vi "45-1523-1 Functional Test.vi"() -> ()   [LabVIEW 2015]
uses:
  <vilib>/DAQmx/write.llb/DAQmx Write (Digital Bool 1Line 1Point).vi
  <vilib>/DAQmx/read.llb/DAQmx Read (Analog DBL 1Chan 1Samp).vi
  Cases.ctl
  <vilib>/ErrorRing/Error Ring.xnode
  <vilib>/LabVIEW Interface for Arduino/LabVIEW Interface for Arduino.lvlib
panel:
  in  "EXIT Button":bool
  in  "Tab Control":T1(tab)
  in  "START Button":bool
  in  "Restart Button":bool
  in  "OK Button":bool
  in  "OK Button 10":bool
  in  "OK Button 3":bool
  in  "OK Button 4":bool
  in  "Restart Button 2":bool
  in  "START Button 2":bool caption="START Button"
  in  "OK Button 5":bool
  in  "OK Button 6":bool
  in  "OK Button 7":bool
  in  "OK Button 8":bool
  in  "OK Button 9":bool
  in  "OK Button 11":bool
  in  "OK Button 12":bool
  # "45-1523-1 Functional Tester"
  # "Click \"START TEST\" To Begin Test"
  # "TESTING J15..."
  # "TESTING K2..."
  # "TESTING K3..."
  # "TESTING K4..."
  # "ALL TESTS PASSED!"
  # "CHECK HIGHLIGHTED CONNECTIONS"
  # "SWITCH K2 FAILED!"
  # "SWITCH K3 FAILED!"
  # "SWITCH K4 FAILED!"
  # "Test Failed"
  # "Verify Connections, then Click \"START\""
  # "Possible Locations of Failure:\n   - Switch K1\n   - S1 Jumper\n   - Q4\n   - U1\n   - Q5"
  # "CHECK HIGHLIGHTED CONNECTIONS"
  # "Power Fault to Board"
  # "CHECK HIGHLIGHTED CONNECTION"
  # "Are All Three LEDs Lit?"
  # "Possible Causes of Failure:\n   - LEDs (Reversed or Faulty)\n   - U1\n   - Q2"
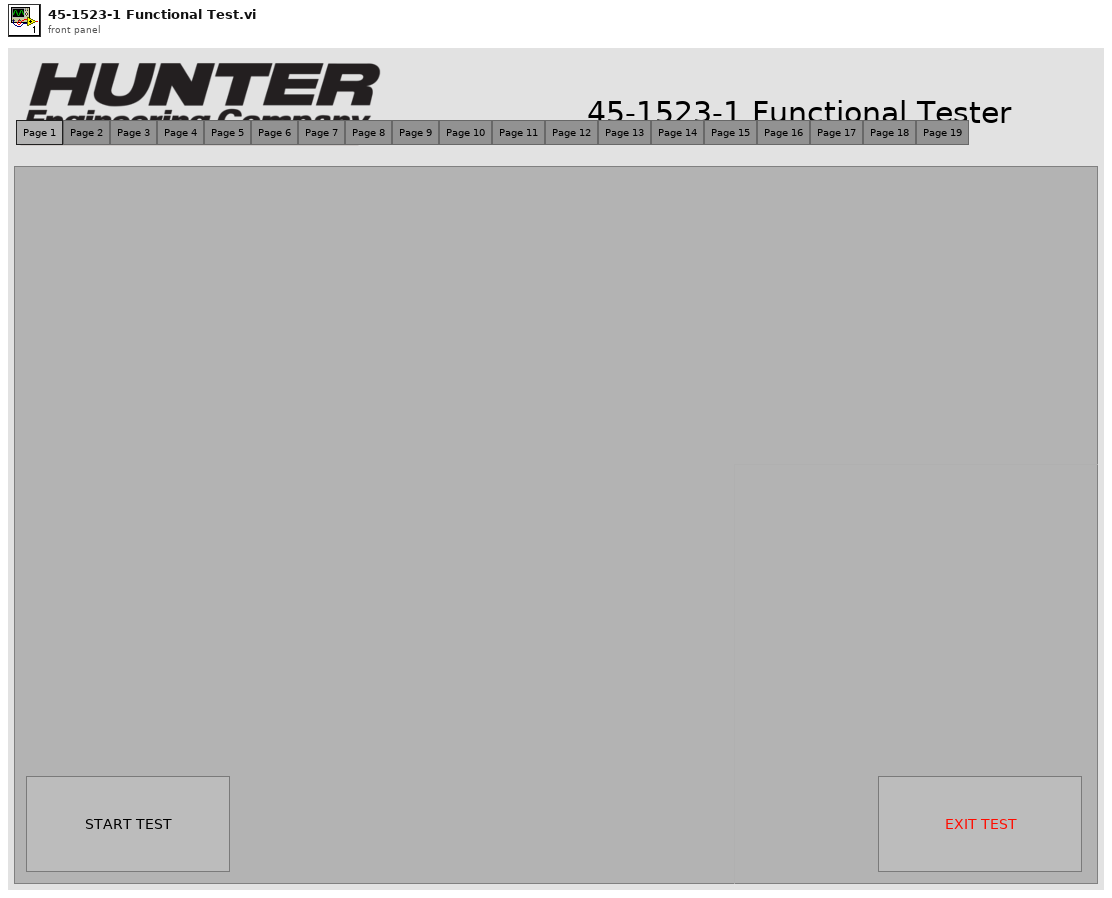
[diagram p1: front panel]
types:
  T1 = enum32{"Page 1", "Page 2", "Page 3", "Page 4", "Page 5", "Page 6", "Page 7", "Page 8", "Page 9", "Page 10", "Page 11", "Page 12", "Page 13", "Page 14", "Page 15", "Page 16", "Page 17", "Page 18", "Page 19"}
  T2 = typedef "Cases.ctl" = enum16{"Start", "Initalization", "J16 Test", "J15 Test", "J15 Error Page", "K2 Test", "K2 Error Page", "K3 Test", "K3 Error Page", "K4 Test", "K4 Error Page", "Test Complete", "Test Failed", "Error", "J15 Failed", "J16 Error", "J16 Failed", "K2 Failed", "LEDs Failed"}
  T3 = typedef "LabVIEW Interface for Arduino.lvlib/Arduino Resource.ctl" = cluster{"VISA resource":refnum<visa-resource-name>, "Board Type":T4, "Connection Type":enum8{"USB / Serial"}, "Bytes Per Packet (15)":u8}
  T4 = typedef "LabVIEW Interface for Arduino.lvlib/Board Type.ctl" = enum16{"Uno", "Dimuelanove w/Atmega 328", "Mega 2560"}
  T5 = enum8{"Enabled", "Disabled", "Disabled and Grayed Out"}
  T6 = enum32{"Page 1", "Page 2", "Page 3", "Page 4", "Page 5", "Page 6", "Page 7", "Page 8", "Page 9", "Page 10", "Page 11"}
  T7 = enum32{"Page 1", "Page 2", "Page 3", "Page 4", "Page 5", "Page 6", "Page 7", "Page 8", "Page 9", "Page 10", "Page 11", "Page 12"}
  T8 = enum32{"Page 1", "Page 2", "Page 3", "Page 4", "Page 5", "Page 6", "Page 7", "Page 8", "Page 9", "Page 10", "Page 11", "Page 12", "Page 13", "Page 14", "Page 15", "Page 16", "Page 17"}
  T9 = enum32{"Page 1", "Page 2", "Page 3", "Page 4", "Page 5", "Page 6", "Page 7", "Page 8", "Page 9", "Page 10", "Page 11", "Page 12", "Page 13", "Page 14", "Page 15", "Page 16", "Page 17", "Page 18"}
  T10 = enum32{"Page 1", "Page 2", "Page 3", "Page 4", "Page 5", "Page 6", "Page 7", "Page 8", "Page 9", "Page 10", "Page 11", "Page 12", "Page 13", "Page 14", "Page 15", "Page 16"}
  T11 = enum32{"Page 1", "Page 2", "Page 3", "Page 4", "Page 5", "Page 6", "Page 7", "Page 8", "Page 9", "Page 10", "Page 11", "Page 12", "Page 13"}
  T12 = enum32{"Page 1", "Page 2", "Page 3", "Page 4", "Page 5", "Page 6", "Page 7", "Page 8", "Page 9", "Page 10", "Page 11", "Page 12", "Page 13", "Page 14"}
  T13 = enum32{"Page 1", "Page 2", "Page 3", "Page 4", "Page 5", "Page 6", "Page 7", "Page 8", "Page 9", "Page 10", "Page 11", "Page 12", "Page 13", "Page 14", "Page 15"}
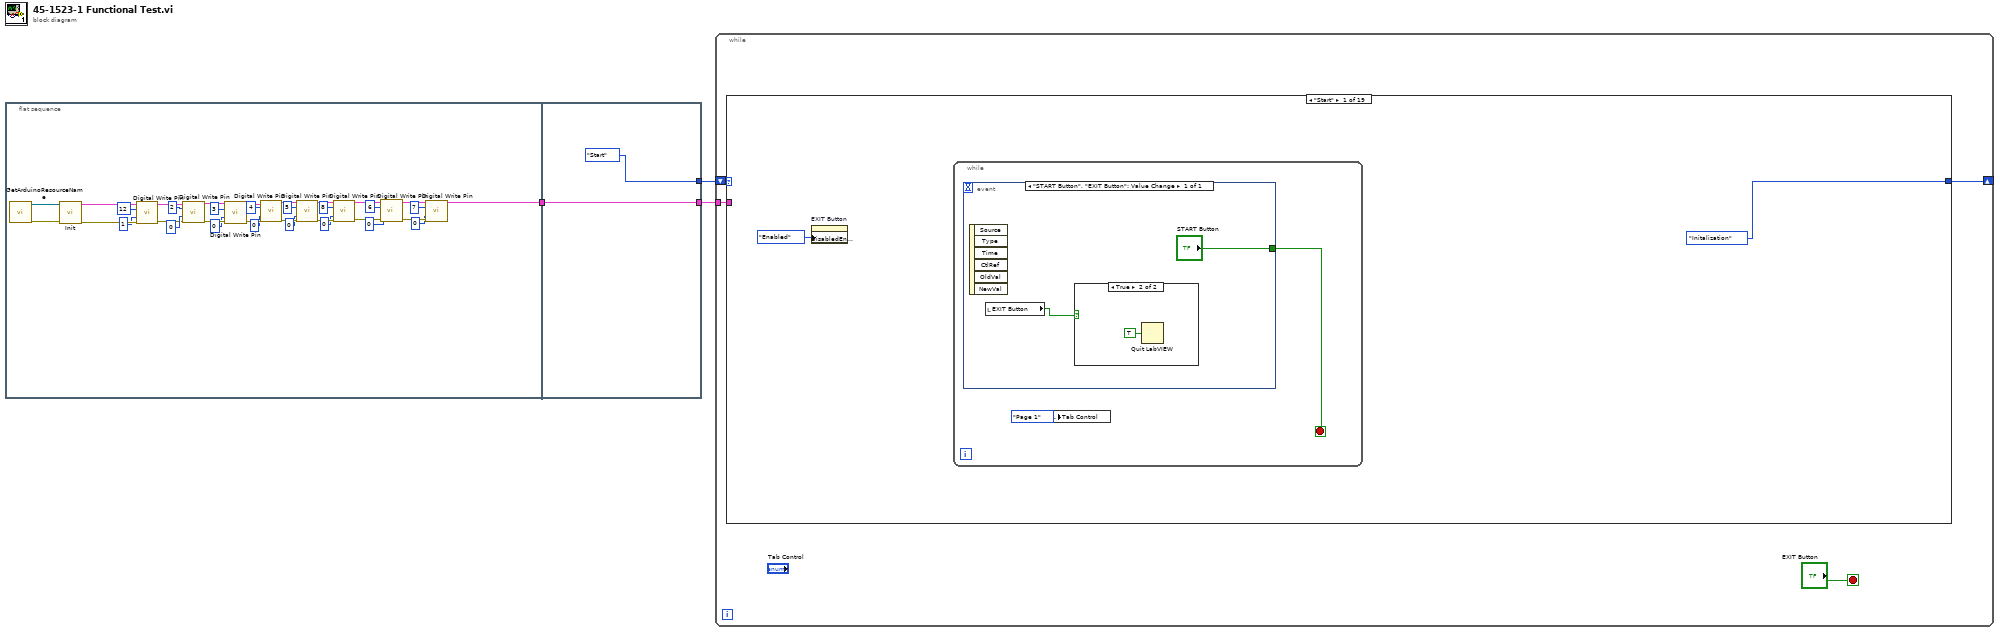
[diagram p0: block diagram]
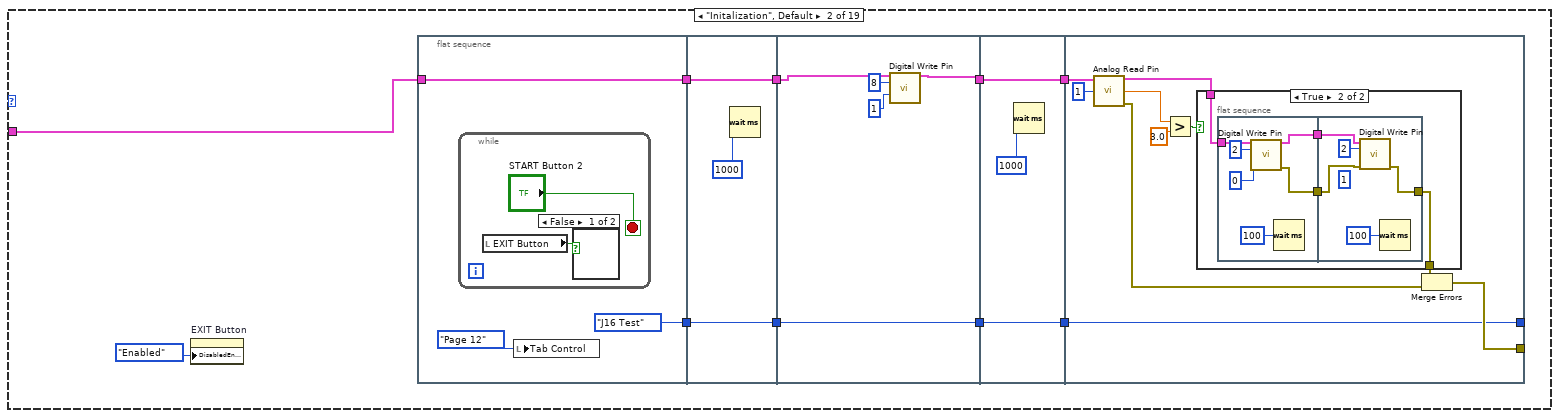
[diagram p3: hidden frame]
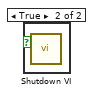
[diagram p4: hidden frame]
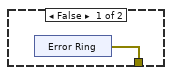
[diagram p5: hidden frame]
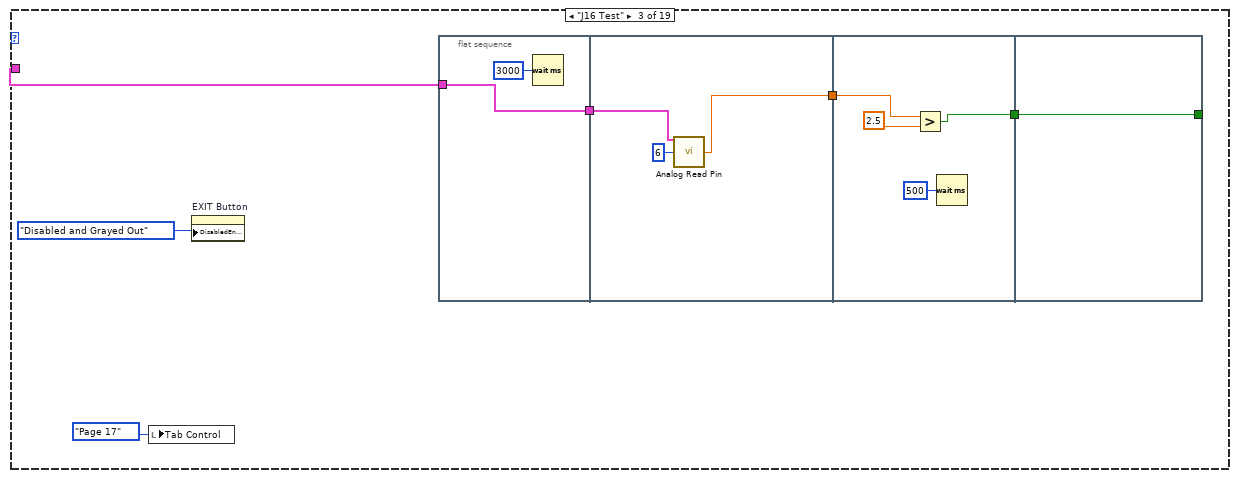
[diagram p6: hidden frame]
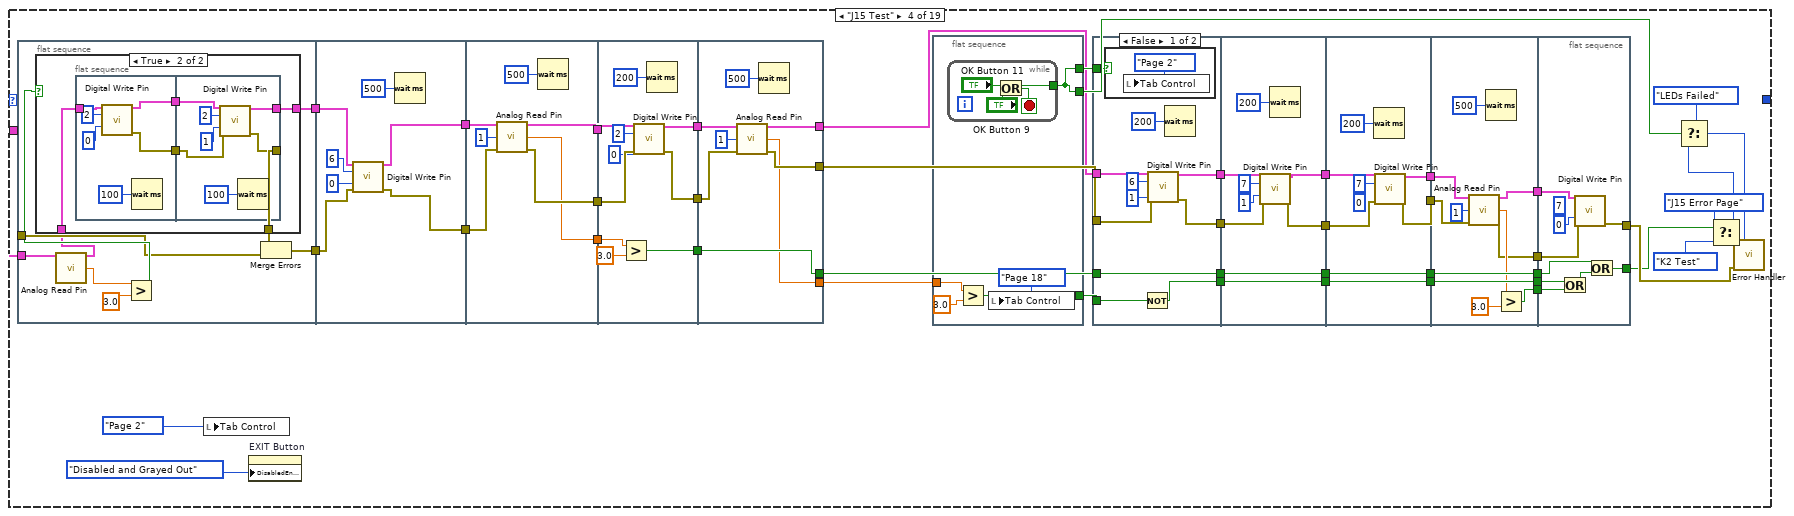
[diagram p7: hidden frame]
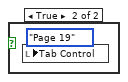
[diagram p8: hidden frame]
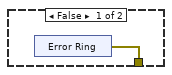
[diagram p9: hidden frame]
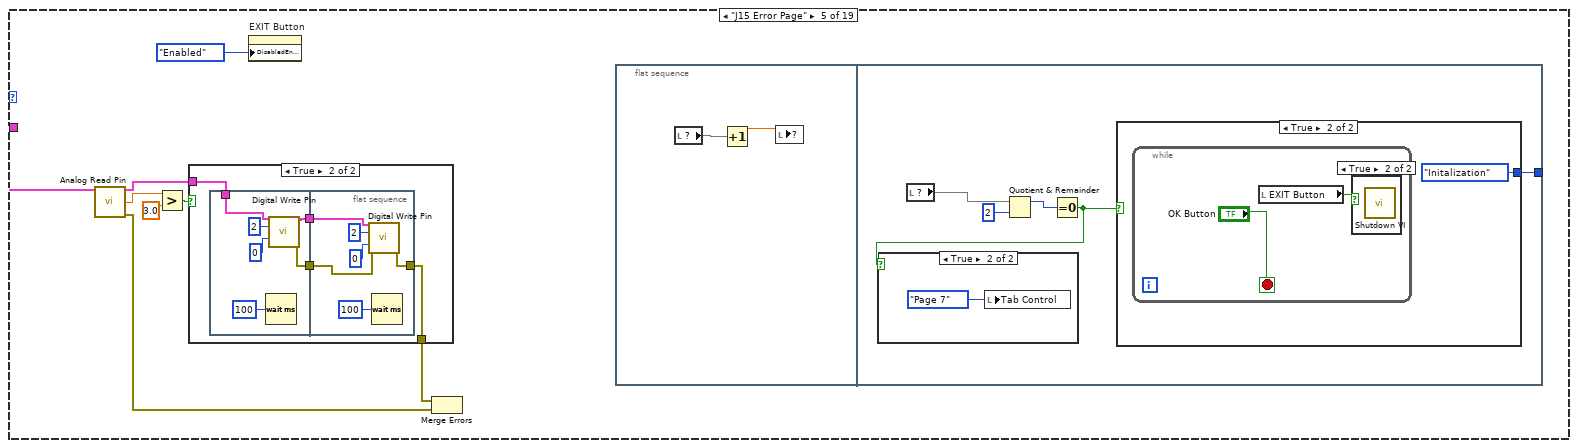
[diagram p10: hidden frame]
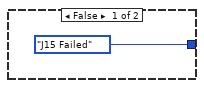
[diagram p12: hidden frame]
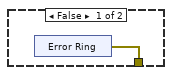
[diagram p14: hidden frame]
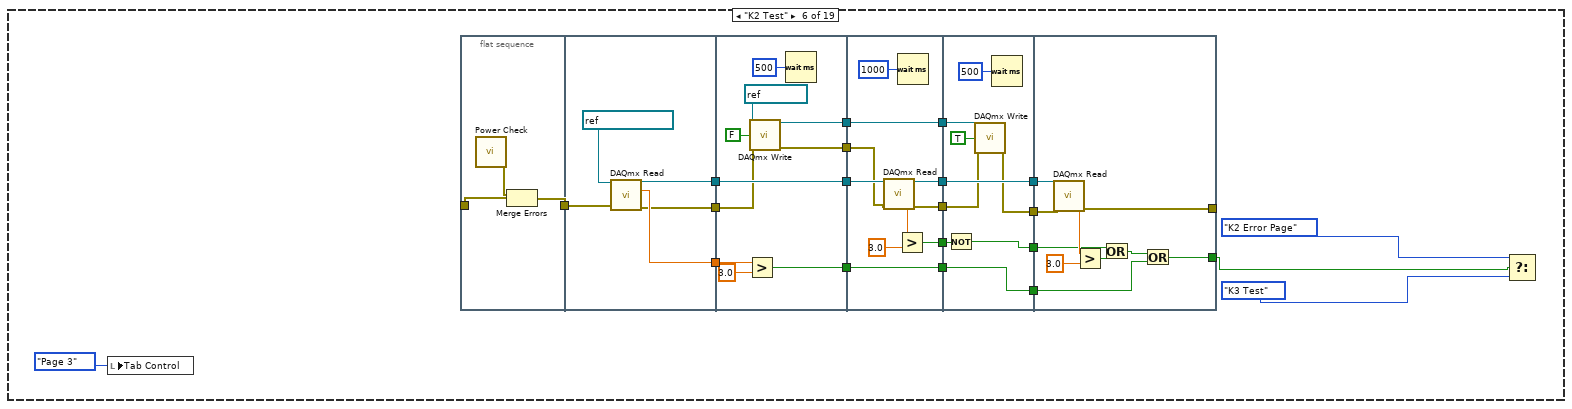
[diagram p15: hidden frame]
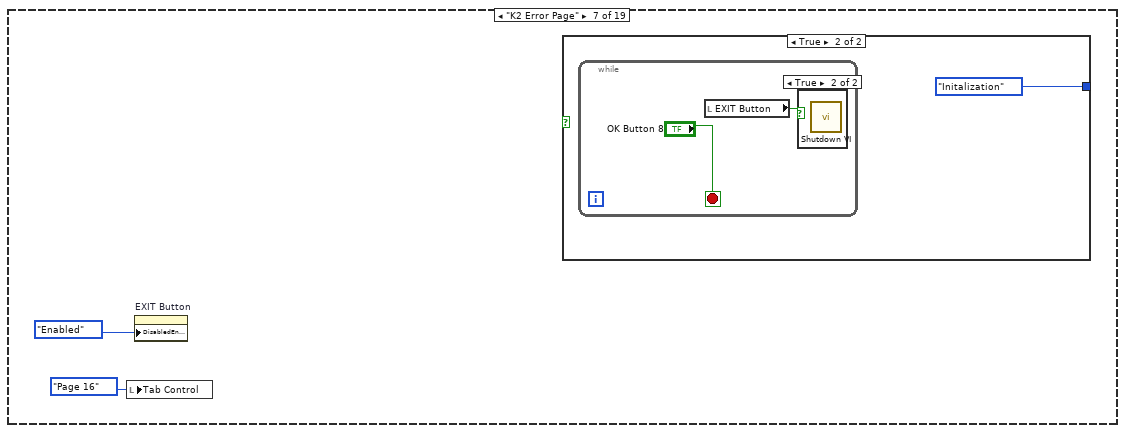
[diagram p16: hidden frame]
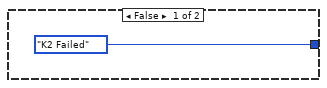
[diagram p17: hidden frame]
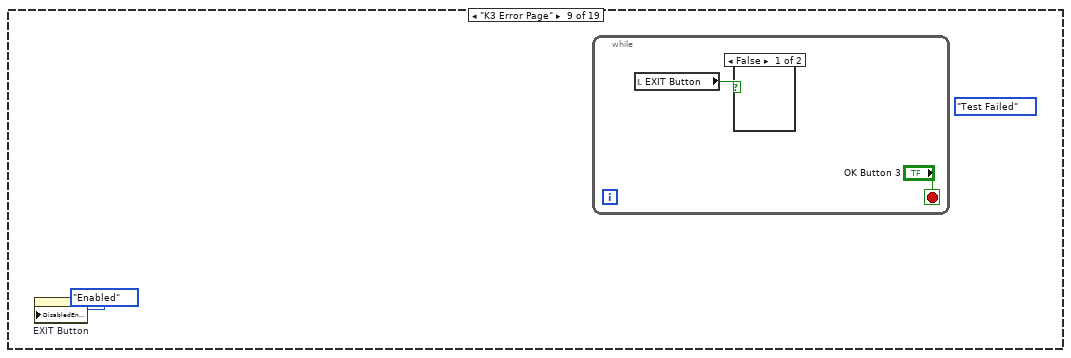
[diagram p20: hidden frame]
diagram:
  n1 = flat-sequence {
    tunnel: [w10] -> w3
    tunnel: [Cases."Start" ("Enum")] -> w1
    tunnel: [w39] -> w2
    tunnel: w3 -> [w39]
    frame #0 {
      n2 = call "GetArduinoResourceName.vi"() -> ("error out"=w37:errorcluster, "VISA resource name"=w38:refnum<visa-resource-name>)  [unwired: 10 in]
      n3 = call <vilib>:"Init.vi"("VISA resource"=w38, "error in"=w37) -> ("Arduino Resource"=w9:T3, "error out"=w8:errorcluster)  [unwired: 16 in]
      n4 = call <vilib>:"Digital Write Pin.vi"("Arduino Resource"=w9, "Digital I/O Pin (0)"=u8 12, "Value (0)"=u8 1, "error in"=w8) -> ("Arduino Resource"=w6:T3, "error out"=w7:errorcluster)  [unwired: 10 in]
      n5 = call <vilib>:"Digital Write Pin.vi"("Arduino Resource"=w6, "Digital I/O Pin (0)"=u8 2, "Value (0)"=u8 0, "error in"=w7) -> ("Arduino Resource"=w36:T3, "error out"=w35:errorcluster)  [unwired: 10 in]
      n6 = call <vilib>:"Digital Write Pin.vi"("Arduino Resource"=w36, "Digital I/O Pin (0)"=u8 3, "Value (0)"=u8 0, "error in"=w35) -> ("Arduino Resource"=w34:T3, "error out"=w33:errorcluster)  [unwired: 10 in]
      n7 = call <vilib>:"Digital Write Pin.vi"("Arduino Resource"=w34, "Digital I/O Pin (0)"=u8 4, "Value (0)"=u8 0, "error in"=w33) -> ("Arduino Resource"=w32:T3, "error out"=w31:errorcluster)  [unwired: 10 in]
      n8 = call <vilib>:"Digital Write Pin.vi"("Arduino Resource"=w32, "Digital I/O Pin (0)"=u8 5, "Value (0)"=u8 0, "error in"=w31) -> ("Arduino Resource"=w30:T3, "error out"=w29:errorcluster)  [unwired: 10 in]
      n9 = call <vilib>:"Digital Write Pin.vi"("Arduino Resource"=w30, "Digital I/O Pin (0)"=u8 8, "Value (0)"=u8 0, "error in"=w29) -> ("Arduino Resource"=w18:T3, "error out"=w15:errorcluster)  [unwired: 10 in]
      n10 = call <vilib>:"Digital Write Pin.vi"("Arduino Resource"=w18, "Digital I/O Pin (0)"=u8 6, "Value (0)"=u8 0, "error in"=w15) -> ("Arduino Resource"=w13:T3, "error out"=w14:errorcluster)  [unwired: 10 in]
      n11 = call <vilib>:"Digital Write Pin.vi"("Arduino Resource"=w13, "Digital I/O Pin (0)"=u8 7, "Value (0)"=u8 0, "error in"=w14) -> ("Arduino Resource"=w10:T3)  [unwired: 10 in, 1 out]
    }
    frame #1 {
    }
  }
  n12 = while {
    tunnel: w2 -> [w43]
    shift-right: [w41] -> _
    shift-left: w1 -> [w42]
    stop <- "EXIT Button" stop-if-true
    n13 = case shown="\"Start\"" w42 {
      tunnel: w43 -> [_ w60 w105 w131 w288 _ _ _ _ _ _ _ _ _ _ _ _ _ _]
      tunnel: [Cases."Initalization" ("Enum") _ _ _ _ _ _ _ _ _ _ _ _ _ _ _ _ _ _] -> w41
      frame "Start" {
        n14 = property on="EXIT Button" class="Bool (strict)"("DisabledEnum"=T5."Enabled" ("Disabled")) -> ()  [unwired: 2 in, 2 out]
        n15 = while {
          stop <- w48 stop-if-true
          n16 = event shown="[0] \"START Button\", \"EXIT Button\": Value Change" {
            selector: _ -> [_]
            dyn-events: _ -> [_]
            timeout: _ -> [_]
            tunnel: ["START Button"] -> w48
            event "START Button", "EXIT Button": Value Change {
              n17 = event-data() -> ()  [unwired: 1 in, 6 out]
              n18 = local read "EXIT Button"() -> (w50:bool)
              n19 = case shown="True" w50 {
                frame False {
                }
                frame True {
                  n20 = Quit LabVIEW(quit? (T)=TRUE) -> ()
                }
              }
            }
          }
          n21 = local write "Tab Control"(T6."Page 1" ("Tab Control")) -> ()
        }
      }
      frame "Initalization", Default {
        n22 = property on="EXIT Button" class="Bool (strict)"("DisabledEnum"=T5."Enabled" ("Disabled")) -> ()  [unwired: 2 in, 2 out]
        n23 = flat-sequence {
          tunnel: [Cases."J16 Test" ("Enum")] -> w59
          tunnel: [w62] -> w57
          tunnel: w60 -> [w62]
          tunnel: w59 -> [w69]
          tunnel: [w69] -> w58
          tunnel: w57 -> [w68]
          tunnel: [w68] -> w56
          tunnel: w58 -> [w74]
          tunnel: [w74] -> w55
          tunnel: w56 -> [w73]
          tunnel: [w72] -> w53
          tunnel: w55 -> [w77]
          tunnel: [w77] -> w54
          tunnel: w53 -> [w76]
          tunnel: [w76] -> w52
          tunnel: w54 -> [w83]
          tunnel: [w84] -> _
          tunnel: [w83] -> _
          tunnel: w52 -> [w80]
          frame #0 {
            n24 = while {
              stop <- "START Button 2" stop-if-true
              n25 = local read "EXIT Button"() -> (w65:bool)
              n26 = case shown="False" w65 {
                frame False {
                }
                frame True {
                  n27 = call "Shutdown VI.vi"() -> ()  [unwired: 12 in]
                }
              }
            }
            n28 = local write "Tab Control"(T7."Page 12" ("Tab Control")) -> ()
          }
          frame #1 {
            n29 = Wait (ms)(milliseconds to wait=u32 1000) -> ()  [unwired: 1 out]
          }
          frame #2 {
            n30 = call <vilib>:"Digital Write Pin.vi"("Arduino Resource"=w73, "Digital I/O Pin (0)"=u8 8, "Value (0)"=u8 1) -> ("Arduino Resource"=w72:T3)  [unwired: 11 in, 1 out]
          }
          frame #3 {
            n31 = Wait (ms)(milliseconds to wait=u32 1000) -> ()  [unwired: 1 out]
          }
          frame #4 {
            n32 = call <vilib>:"Analog Read Pin.vi"("Arduino Resource"=w80, "Analog Input Pin (0)"=u8 1) -> ("Arduino Resource"=w78:T3, "Voltage"=w82:dbl, "error out"=w81:errorcluster)  [unwired: 11 in]
            n33 = Greater?(x=w82, y=3.0) -> (0:w86:bool)
            n34 = case shown="True" w86 {
              tunnel: [w88 w92] -> w85
              tunnel: w78 -> [_ w91]
              frame False {
                n35 = xnode "Error Ring"() -> ("error out"=w88:errorcluster)
              }
              frame True {
                n36 = flat-sequence {
                  tunnel: [w96] -> w93
                  tunnel: w91 -> [w98]
                  tunnel: [w94] -> w90
                  tunnel: [w101] -> w92
                  tunnel: w93 -> [w102]
                  tunnel: w90 -> [w100]
                  frame #0 {
                    n37 = call <vilib>:"Digital Write Pin.vi"("Arduino Resource"=w98, "Digital I/O Pin (0)"=u8 2, "Value (0)"=u8 0) -> ("Arduino Resource"=w94:T3, "error out"=w96:errorcluster)  [unwired: 11 in]
                    n38 = Wait (ms)(milliseconds to wait=u32 100) -> ()  [unwired: 1 out]
                  }
                  frame #1 {
                    (unwired) u8 1 ("Value (0)")
                    n39 = call <vilib>:"Digital Write Pin.vi"("Arduino Resource"=w100, "Digital I/O Pin (0)"=u8 2, "error in"=w102) -> ("error out"=w101:errorcluster)  [unwired: 11 in, 1 out]
                    n40 = Wait (ms)(milliseconds to wait=u32 100) -> ()  [unwired: 1 out]
                  }
                }
              }
            }
            n41 = Merge Errors(w85, w81) -> (w84:errorcluster)
          }
        }
      }
      frame "J16 Test" {
        n42 = local write "Tab Control"(T8."Page 17" ("Tab Control")) -> ()
        n43 = property on="EXIT Button" class="Bool (strict)"("DisabledEnum"=T5."Disabled and Grayed Out" ("Disabled")) -> ()  [unwired: 2 in, 2 out]
        n44 = flat-sequence {
          tunnel: [w111] -> w106
          tunnel: w105 -> [w111]
          tunnel: [w115] -> w110
          tunnel: w106 -> [w114]
          tunnel: w110 -> [w117]
          tunnel: [w116] -> w108
          tunnel: [w120] -> _
          tunnel: w108 -> [w120]
          frame #0 {
            n45 = Wait (ms)(milliseconds to wait=u32 3000) -> ()  [unwired: 1 out]
          }
          frame #1 {
            n46 = call <vilib>:"Analog Read Pin.vi"("Arduino Resource"=w114, "Analog Input Pin (0)"=u8 6) -> ("Voltage"=w115:dbl)  [unwired: 11 in, 2 out]
          }
          frame #2 {
            n47 = Greater?(x=w117, y=2.5) -> (0:w116:bool)
            n48 = Wait (ms)(milliseconds to wait=u32 500) -> ()  [unwired: 1 out]
          }
          frame #3 {
          }
        }
      }
      frame "J15 Test" {
        n49 = flat-sequence {
          tunnel: [w232] -> w161
          tunnel: w131 -> [w229]
          tunnel: [w227] -> w130
          tunnel: [w226] -> w129
          tunnel: [w260] -> w164
          tunnel: w130 -> [w259]
          tunnel: w129 -> [w258]
          tunnel: [w255] -> w128
          tunnel: [w264] -> w165
          tunnel: w164 -> [w266]
          tunnel: [w267] -> w163
          tunnel: w128 -> [w265]
          tunnel: [w262] -> w127
          tunnel: w165 -> [w277]
          tunnel: w163 -> [w273]
          tunnel: [w274] -> w162
          tunnel: [w275] -> w158
          tunnel: w127 -> [w272]
          tunnel: [w269] -> w126
          tunnel: w162 -> [w284]
          tunnel: w158 -> [w285]
          tunnel: [w285] -> w155
          tunnel: [w283] -> w144
          tunnel: [w282] -> w135
          tunnel: w126 -> [w281]
          tunnel: [w279] -> w125
          frame #0 {
            n50 = call <vilib>:"Analog Read Pin.vi"("Arduino Resource"=w229) -> ("Arduino Resource"=w228:T3, "Voltage"=w230:dbl)  [unwired: 12 in, 1 out]
            n51 = Greater?(x=w230, y=3.0) -> (0:w234:bool)
            n52 = case shown="True" w234 {
              tunnel: [w235 w240] -> w233
              tunnel: w228 -> [_ w239]
              tunnel: [_ w237] -> w226
              frame False {
                n53 = xnode "Error Ring"() -> ("error out"=w235:errorcluster)
              }
              frame True {
                n54 = flat-sequence {
                  tunnel: [w246] -> w241
                  tunnel: w239 -> [w245]
                  tunnel: [w242] -> w238
                  tunnel: [w250] -> w240
                  tunnel: w241 -> [w251]
                  tunnel: w238 -> [w249]
                  tunnel: [w248] -> w237
                  frame #0 {
                    n55 = call <vilib>:"Digital Write Pin.vi"("Arduino Resource"=w245, "Digital I/O Pin (0)"=u8 2, "Value (0)"=u8 0) -> ("Arduino Resource"=w242:T3, "error out"=w246:errorcluster)  [unwired: 11 in]
                    n56 = Wait (ms)(milliseconds to wait=u32 100) -> ()  [unwired: 1 out]
                  }
                  frame #1 {
                    n57 = call <vilib>:"Digital Write Pin.vi"("Arduino Resource"=w249, "Digital I/O Pin (0)"=u8 2, "Value (0)"=u8 1, "error in"=w251) -> ("Arduino Resource"=w248:T3, "error out"=w250:errorcluster)  [unwired: 10 in]
                    n58 = Wait (ms)(milliseconds to wait=u32 100) -> ()  [unwired: 1 out]
                  }
                }
              }
            }
            n59 = Merge Errors(w233, w232) -> (w227:errorcluster)
          }
          frame #1 {
            n60 = call <vilib>:"Digital Write Pin.vi"("Arduino Resource"=w258, "Digital I/O Pin (0)"=u8 6, "Value (0)"=u8 0, "error in"=w259) -> ("Arduino Resource"=w255:T3, "error out"=w260:errorcluster)  [unwired: 10 in]
            n61 = Wait (ms)(milliseconds to wait=u32 500) -> ()  [unwired: 1 out]
          }
          frame #2 {
            n62 = call <vilib>:"Analog Read Pin.vi"("Arduino Resource"=w265, "Analog Input Pin (0)"=u8 1, "error in"=w266) -> ("Arduino Resource"=w262:T3, "Voltage"=w264:dbl, "error out"=w267:errorcluster)  [unwired: 10 in]
            n63 = Wait (ms)(milliseconds to wait=u32 500) -> ()  [unwired: 1 out]
          }
          frame #3 {
            n64 = Greater?(x=w277, y=3.0) -> (0:w275:bool)
            n65 = call <vilib>:"Digital Write Pin.vi"("Arduino Resource"=w272, "Digital I/O Pin (0)"=u8 2, "Value (0)"=u8 0, "error in"=w273) -> ("Arduino Resource"=w269:T3, "error out"=w274:errorcluster)  [unwired: 10 in]
            n66 = Wait (ms)(milliseconds to wait=u32 200) -> ()  [unwired: 1 out]
          }
          frame #4 {
            n67 = call <vilib>:"Analog Read Pin.vi"("Arduino Resource"=w281, "Analog Input Pin (0)"=u8 1, "error in"=w284) -> ("Arduino Resource"=w279:T3, "Voltage"=w282:dbl, "error out"=w283:errorcluster)  [unwired: 10 in]
            n68 = Wait (ms)(milliseconds to wait=u32 500) -> ()  [unwired: 1 out]
          }
        }
        n69 = local write "Tab Control"(T6."Page 2" ("Tab Control")) -> ()
        n70 = property on="EXIT Button" class="Bool (strict)"("DisabledEnum"=T5."Disabled and Grayed Out" ("Disabled")) -> ()  [unwired: 2 in, 2 out]
        n71 = flat-sequence {
          tunnel: w135 -> [w171]
          tunnel: [w170] -> w134
          tunnel: [w168] -> w133
          tunnel: [w168] -> w132
          frame #0 {
            n72 = while {
              tunnel: ["OK Button 11"] -> w168
              stop <- w173 stop-if-true
              n73 = Or(x="OK Button 11", y="OK Button 9") -> (x .or. y?=w173:bool)
            }
            n74 = Greater?(x=w171, y=3.0) -> (0:w170:bool)
            n75 = local write "Tab Control"(T9."Page 18" ("Tab Control")) -> ()
          }
        }
        n76 = flat-sequence {
          tunnel: w134 -> [w185]
          tunnel: w155 -> [w184]
          tunnel: [w184] -> w151
          tunnel: [w183] -> w150
          tunnel: w144 -> [w181]
          tunnel: [w180] -> w143
          tunnel: w132 -> [w182]
          tunnel: w125 -> [w179]
          tunnel: [w176] -> w124
          tunnel: [w196] -> w152
          tunnel: w151 -> [w196]
          tunnel: w150 -> [w195]
          tunnel: [w195] -> w149
          tunnel: w143 -> [w194]
          tunnel: [w193] -> w142
          tunnel: w124 -> [w192]
          tunnel: [w189] -> w123
          tunnel: [w204] -> w153
          tunnel: w152 -> [w204]
          tunnel: w149 -> [w203]
          tunnel: [w203] -> w148
          tunnel: [w201] -> w145
          tunnel: w142 -> [w199]
          tunnel: w123 -> [w200]
          tunnel: [w198] -> w121
          tunnel: [w214] -> w154
          tunnel: w153 -> [w214]
          tunnel: w148 -> [w213]
          tunnel: [w213] -> w147
          tunnel: [w212] -> w146
          tunnel: w145 -> [w208]
          tunnel: [w209] -> w141
          tunnel: [w207] -> w122
          tunnel: w121 -> [w206]
          tunnel: w154 -> [w224]
          tunnel: w147 -> [w223]
          tunnel: w146 -> [w222]
          tunnel: w141 -> [w218]
          tunnel: [w219] -> w140
          tunnel: [w221] -> w136
          tunnel: w122 -> [w217]
          frame #0 {
            n77 = case shown="False" w182 {
              frame False {
                n78 = local write "Tab Control"(T9."Page 2" ("Tab Control")) -> ()
              }
              frame True {
                n79 = local write "Tab Control"(T1."Page 19" ("Tab Control")) -> ()
              }
            }
            n80 = Not(x=w185) -> (.not. x?=w183:bool)
            n81 = call <vilib>:"Digital Write Pin.vi"("Arduino Resource"=w179, "Digital I/O Pin (0)"=u8 6, "Value (0)"=u8 1, "error in"=w181) -> ("Arduino Resource"=w176:T3, "error out"=w180:errorcluster)  [unwired: 10 in]
            n82 = Wait (ms)(milliseconds to wait=u32 200) -> ()  [unwired: 1 out]
          }
          frame #1 {
            n83 = call <vilib>:"Digital Write Pin.vi"("Arduino Resource"=w192, "Digital I/O Pin (0)"=u8 7, "Value (0)"=u8 1, "error in"=w194) -> ("Arduino Resource"=w189:T3, "error out"=w193:errorcluster)  [unwired: 10 in]
            n84 = Wait (ms)(milliseconds to wait=u32 200) -> ()  [unwired: 1 out]
          }
          frame #2 {
            (unwired) u8 0 ("Value (0)")
            n85 = Wait (ms)(milliseconds to wait=u32 200) -> ()  [unwired: 1 out]
            n86 = call <vilib>:"Digital Write Pin.vi"("Arduino Resource"=w200, "Digital I/O Pin (0)"=u8 7, "error in"=w199) -> ("Arduino Resource"=w198:T3, "error out"=w201:errorcluster)  [unwired: 11 in]
          }
          frame #3 {
            n87 = call <vilib>:"Analog Read Pin.vi"("Arduino Resource"=w206, "Analog Input Pin (0)"=u8 1, "error in"=w208) -> ("Arduino Resource"=w207:T3, "Voltage"=w210:dbl, "error out"=w209:errorcluster)  [unwired: 10 in]
            n88 = Wait (ms)(milliseconds to wait=u32 500) -> ()  [unwired: 1 out]
            n89 = Greater?(x=w210, y=3.0) -> (0:w212:bool)
          }
          frame #4 {
            (unwired) u8 7 ("Digital I/O Pin (0)")
            n90 = Or(x=w223, y=w222) -> (x .or. y?=w225:bool)
            n91 = call <vilib>:"Digital Write Pin.vi"("Arduino Resource"=w217, "Value (0)"=u8 0, "error in"=w218) -> ("error out"=w219:errorcluster)  [unwired: 11 in, 1 out]
            n92 = Or(x=w224, y=w225) -> (x .or. y?=w221:bool)
          }
        }
        n93 = Select(t=Cases."J15 Error Page" ("Enum"), s=w136, f=Cases."K2 Test" ("Enum")) -> (s? t:f=w137:T2)
        n94 = Select(t=Cases."LEDs Failed" ("Enum"), s=w133, f=w137) -> (s? t:f=w157:T2)
        n95 = call "Error Handler.vi"("error in (no error)"=w140, "Enum in"=w157) -> ("error out"=w160:errorcluster, "Enum out"=w159:T2)  [unwired: 8 in]
      }
      frame "J15 Error Page" {
        n96 = call <vilib>:"Analog Read Pin.vi"("Arduino Resource"=w288) -> ("Arduino Resource"=w287:T3, "Voltage"=w289:dbl, "error in"=w291:errorcluster, "error out"=w290:errorcluster)  [unwired: 11 in]
        n97 = Greater?(x=w289, y=3.0) -> (0:w293:bool)
        n98 = case shown="True" w293 {
          tunnel: [w308 w312] -> w292
          tunnel: w287 -> [_ w311]
          frame False {
            n99 = xnode "Error Ring"() -> ("error out"=w308:errorcluster)
          }
          frame True {
            n100 = flat-sequence {
              tunnel: [w315] -> w313
              tunnel: w311 -> [w316]
              tunnel: [w314] -> w310
              tunnel: [w321] -> w312
              tunnel: w313 -> [w322]
              tunnel: w310 -> [w320]
              frame #0 {
                n101 = Wait (ms)(milliseconds to wait=u32 100) -> ()  [unwired: 1 out]
                n102 = call <vilib>:"Digital Write Pin.vi"("Arduino Resource"=w316, "Digital I/O Pin (0)"=u8 2, "Value (0)"=u8 0) -> ("Arduino Resource"=w314:T3, "error out"=w315:errorcluster)  [unwired: 11 in]
              }
              frame #1 {
                n103 = call <vilib>:"Digital Write Pin.vi"("Arduino Resource"=w320, "Digital I/O Pin (0)"=u8 2, "Value (0)"=u8 0, "error in"=w322) -> ("error out"=w321:errorcluster)  [unwired: 10 in, 1 out]
                n104 = Wait (ms)(milliseconds to wait=u32 100) -> ()  [unwired: 1 out]
              }
            }
          }
        }
        n105 = property on="EXIT Button" class="Bool (strict)"("DisabledEnum"=T5."Enabled" ("Disabled")) -> ()  [unwired: 2 in, 2 out]
        n106 = Merge Errors(w292, w290) -> ()  [unwired: 1 out]
        n107 = flat-sequence {
          tunnel: [w299] -> _
          frame #0 {
            n108 = local read item#-1() -> (w296)
            n109 = Increment(x=w296) -> (x+1=w297:dbl)
            n110 = local write item#-1(w297) -> ()
          }
          frame #1 {
            n111 = local read item#-1() -> (w301)
            n112 = Quotient & Remainder(x=w301, y=2) -> (x-y*floor(x/y)=w300:i32)  [unwired: 1 out]
            n113 = Equal To 0?(x=w300) -> (x = 0?=w298:bool)
            n114 = case shown="True" w298 {
              frame False {
              }
              frame True {
                n115 = local write "Tab Control"(T6."Page 7" ("Tab Control")) -> ()
              }
            }
            n116 = case shown="True" w298 {
              tunnel: [Cases."J15 Failed" ("Enum") Cases."Initalization" ("Enum")] -> w299
              frame False {
              }
              frame True {
                n117 = while {
                  stop <- "OK Button" stop-if-true
                  n118 = local read "EXIT Button"() -> (w306:bool)
                  n119 = case shown="True" w306 {
                    frame False {
                    }
                    frame True {
                      n120 = call "Shutdown VI.vi"() -> ()  [unwired: 12 in]
                    }
                  }
                }
              }
            }
          }
        }
      }
      frame "K2 Test" {
        n121 = local write "Tab Control"(T6."Page 3" ("Tab Control")) -> ()
        n122 = flat-sequence {
          tunnel: [w350] -> w334
          tunnel: [w348] -> w326
          tunnel: [w354] -> w344
          tunnel: [w353] -> w340
          tunnel: [w351] -> w333
          tunnel: w326 -> [w352]
          tunnel: [w363] -> w347
          tunnel: w344 -> [w362]
          tunnel: [w362] -> w343
          tunnel: w340 -> [w361]
          tunnel: [w356] -> w335
          tunnel: w333 -> [w358]
          tunnel: [w357] -> w332
          tunnel: [w374] -> w346
          tunnel: w347 -> [w374]
          tunnel: w343 -> [w373]
          tunnel: [w372] -> w341
          tunnel: [w369] -> w339
          tunnel: [w368] -> w336
          tunnel: w335 -> [w368]
          tunnel: w332 -> [w367]
          tunnel: [w366] -> w331
          tunnel: w346 -> [w383]
          tunnel: [w381] -> w342
          tunnel: w341 -> [w381]
          tunnel: w339 -> [w380]
          tunnel: [w376] -> w338
          tunnel: [w379] -> w337
          tunnel: w336 -> [w379]
          tunnel: w331 -> [w378]
          tunnel: [w377] -> w330
          tunnel: [w390] -> w329
          tunnel: w342 -> [w394]
          tunnel: w338 -> [w391]
          tunnel: w337 -> [w388]
          tunnel: w330 -> [w387]
          tunnel: [w386] -> _
          frame #0 {
            n123 = call "Power Check.vi"() -> ("error out"=w349:errorcluster)  [unwired: 11 in]
            n124 = Merge Errors(w349, w350) -> (w348:errorcluster)
          }
          frame #1 {
            n125 = call-poly <vilib>:"DAQmx Read.vi"("task/channels in"=refnum<k21> "Is K2 Closed", "error in"=w352) -> ("task out"=w354:refnum<k21>, "data"=w353:dbl, "error out"=w351:errorcluster)  [unwired: 11 in]
          }
          frame #2 {
            n126 = Greater?(x=w361, y=3.0) -> (0:w356:bool)
            n127 = call-poly <vilib>:"DAQmx Write.vi"("task/channels in"=refnum<k21> "Fire K2" ("DAQmx Task Name"), "data"=FALSE, "error in"=w358) -> ("task out"=w363:refnum<k21>, "error out"=w357:errorcluster)  [unwired: 10 in, 1 out]
            n128 = Wait (ms)(milliseconds to wait=u32 500) -> ()  [unwired: 1 out]
          }
          frame #3 {
            n129 = call-poly <vilib>:"DAQmx Read.vi"("task/channels in"=w373, "error in"=w367) -> ("task out"=w372:refnum<k21>, "data"=w370:dbl, "error out"=w366:errorcluster)  [unwired: 11 in]
            n130 = Greater?(x=w370, y=3.0) -> (0:w369:bool)
            n131 = Wait (ms)(milliseconds to wait=u32 1000) -> ()  [unwired: 1 out]
          }
          frame #4 {
            n132 = Not(x=w380) -> (.not. x?=w376:bool)
            n133 = call-poly <vilib>:"DAQmx Write.vi"("task/channels in"=w383, "data"=TRUE, "error in"=w378) -> ("error out"=w377:errorcluster)  [unwired: 10 in, 2 out]
            n134 = Wait (ms)(milliseconds to wait=u32 500) -> ()  [unwired: 1 out]
          }
          frame #5 {
            n135 = call-poly <vilib>:"DAQmx Read.vi"("task/channels in"=w394, "error in"=w387) -> ("data"=w392:dbl, "error out"=w386:errorcluster)  [unwired: 11 in, 1 out]
            n136 = Greater?(x=w392, y=3.0) -> (0:w385:bool)
            n137 = Or(x=w391, y=w385) -> (x .or. y?=w389:bool)
            n138 = Or(x=w389, y=w388) -> (x .or. y?=w390:bool)
          }
        }
        n139 = Select(t=Cases."K2 Error Page" ("Enum"), s=w329, f=Cases."K3 Test" ("Enum")) -> ()  [unwired: 1 out]
      }
      frame "K2 Error Page" {
        n140 = local write "Tab Control"(T10."Page 16" ("Tab Control")) -> ()
        n141 = property on="EXIT Button" class="Bool (strict)"("DisabledEnum"=T5."Enabled" ("Disabled")) -> ()  [unwired: 2 in, 2 out]
        n142 = case shown="True" {
          selector: _ -> [_ _]
          tunnel: [Cases."K2 Failed" ("Enum") Cases."Initalization" ("Enum")] -> _
          frame False {
          }
          frame True {
            n143 = while {
              stop <- "OK Button 8" stop-if-true
              n144 = local read "EXIT Button"() -> (w399:bool)
              n145 = case shown="True" w399 {
                frame False {
                }
                frame True {
                  n146 = call "Shutdown VI.vi"() -> ()  [unwired: 12 in]
                }
              }
            }
          }
        }
      }
      frame "K3 Test" {
      }
      frame "K3 Error Page" {
        (unwired) Cases."Test Failed" ("Enum")
        n147 = property on="EXIT Button" class="Bool (strict)"("DisabledEnum"=T5."Enabled" ("Disabled")) -> ()  [unwired: 2 in, 2 out]
        n148 = while {
          stop <- "OK Button 3" stop-if-true
          n149 = local read "EXIT Button"() -> (w402:bool)
          n150 = case shown="False" w402 {
            frame False {
            }
            frame True {
              n151 = call "Shutdown VI.vi"() -> ()  [unwired: 12 in]
            }
          }
        }
      }
      frame "K4 Test" {
      }
      frame "K4 Error Page" {
        (unwired) Cases."Test Failed" ("Enum")
        n152 = local write "Tab Control"(T6."Page 10" ("Tab Control")) -> ()
        n153 = property on="EXIT Button" class="Bool (strict)"("DisabledEnum"=T5."Enabled" ("Disabled")) -> ()  [unwired: 2 in, 2 out]
        n154 = while {
          stop <- "OK Button 4" stop-if-true
          n155 = local read "EXIT Button"() -> (w406:bool)
          n156 = case shown="True" w406 {
            frame False {
            }
            frame True {
              n157 = call "Shutdown VI.vi"() -> ()  [unwired: 12 in]
            }
          }
        }
      }
      frame "Test Complete" {
        n158 = local write "Tab Control"(T6."Page 6" ("Tab Control")) -> ()
        n159 = property on="EXIT Button" class="Bool (strict)"("DisabledEnum"=T5."Enabled" ("Disabled")) -> ()  [unwired: 2 in, 2 out]
        n160 = event shown="[0] \"Restart Button\", \"EXIT Button\": Value Change" {
          selector: _ -> [_]
          dyn-events: _ -> [_]
          timeout: _ -> [_]
          tunnel: [Cases."Start" ("Enum")] -> _
          event "Restart Button", "EXIT Button": Value Change {
            n161 = event-data() -> ()  [unwired: 1 in, 6 out]
            n162 = while {
              stop <- "Restart Button" stop-if-true
              n163 = local read "EXIT Button"() -> (w411:bool)
              n164 = case shown="True" w411 {
                frame False {
                }
                frame True {
                  n165 = call "Shutdown VI.vi"() -> ()  [unwired: 12 in]
                }
              }
            }
          }
        }
      }
      frame "Test Failed" {
        (unwired) Cases."Start" ("Enum")
        n166 = local write "Tab Control"(T6."Page 11" ("Tab Control")) -> ()
        n167 = call-poly <vilib>:"DAQmx Read.vi"("task/channels in"=refnum<k21> "Is J15 Closed") -> ("data"=w417:dbl, "error out"=w413:errorcluster)  [unwired: 12 in, 1 out]
        n168 = Greater?(x=w417, y=3.0) -> (0:w415:bool)
        n169 = case shown="True" w415 {
          tunnel: [w420 w422] -> w414
          frame False {
            n170 = xnode "Error Ring"() -> ("error out"=w420:errorcluster)
          }
          frame True {
            n171 = flat-sequence {
              tunnel: [w426] -> w423
              tunnel: [w431] -> w422
              tunnel: w423 -> [w432]
              frame #0 {
                n172 = call-poly <vilib>:"DAQmx Write.vi"("task/channels in"=refnum<k21> "Fire K1", "data"=FALSE) -> ("error out"=w426:errorcluster)  [unwired: 11 in, 2 out]
                n173 = Wait (ms)(milliseconds to wait=u32 100) -> ()  [unwired: 1 out]
              }
              frame #1 {
                n174 = call-poly <vilib>:"DAQmx Write.vi"("task/channels in"=refnum<k21> "Fire K1", "data"=TRUE, "error in"=w432) -> ("error out"=w431:errorcluster)  [unwired: 10 in, 2 out]
                n175 = Wait (ms)(milliseconds to wait=u32 100) -> ()  [unwired: 1 out]
              }
            }
          }
        }
        n176 = Merge Errors(w414, w413) -> ()  [unwired: 1 in, 1 out]
        n177 = event shown="[0] \"EXIT Button\", \"Restart Button 2\": Value Change" {
          selector: _ -> [_]
          dyn-events: _ -> [_]
          timeout: _ -> [_]
          event "EXIT Button", "Restart Button 2": Value Change {
            n178 = event-data() -> ()  [unwired: 1 in, 6 out]
            n179 = while {
              stop <- "Restart Button 2" stop-if-true
              n180 = local read "EXIT Button"() -> (w433:bool)
              n181 = case shown="False" w433 {
                frame False {
                }
                frame True {
                  n182 = call "Shutdown VI.vi"() -> ()  [unwired: 12 in]
                }
              }
            }
          }
        }
      }
      frame "Error" {
      }
      frame "J15 Failed" {
        n183 = local write "Tab Control"(T11."Page 13" ("Tab Control")) -> ()
        n184 = property on="EXIT Button" class="Bool (strict)"("DisabledEnum"=T5."Enabled" ("Disabled")) -> ()  [unwired: 2 in, 2 out]
        n185 = while {
          stop <- "OK Button 5" stop-if-true
          n186 = local read "EXIT Button"() -> (w437:bool)
          n187 = case shown="True" w437 {
            frame False {
            }
            frame True {
              n188 = call "Shutdown VI.vi"() -> ()  [unwired: 12 in]
            }
          }
        }
      }
      frame "J16 Error" {
        n189 = while {
          stop <- TRUE stop-if-true
          n190 = local read item#-1() -> (w446)
          n191 = Increment(x=w446) -> (x+1=w445:dbl)
          n192 = local write item#-1(w445) -> ()
        }
        n193 = local write "Tab Control"(T12."Page 14" ("Tab Control")) -> ()
        n194 = property on="EXIT Button" class="Bool (strict)"("DisabledEnum"=T5."Enabled" ("Disabled")) -> ()  [unwired: 2 in, 2 out]
        n195 = case shown="True" {
          selector: _ -> [_ _]
          tunnel: [Cases."J16 Failed" ("Enum") Cases."Initalization" ("Enum")] -> _
          frame False {
          }
          frame True {
            n196 = while {
              stop <- "OK Button 6" stop-if-true
              n197 = local read "EXIT Button"() -> (w443:bool)
              n198 = case shown="False" w443 {
                frame False {
                }
                frame True {
                  n199 = call "Shutdown VI.vi"() -> ()  [unwired: 12 in]
                }
              }
            }
          }
        }
      }
      frame "J16 Failed" {
        (unwired) Cases."Test Failed" ("Enum")
        n200 = local write "Tab Control"(T13."Page 15" ("Tab Control")) -> ()
        n201 = property on="EXIT Button" class="Bool (strict)"("DisabledEnum"=T5."Enabled" ("Disabled")) -> ()  [unwired: 2 in, 2 out]
        n202 = while {
          stop <- "OK Button 7" stop-if-true
          n203 = local read "EXIT Button"() -> (w450:bool)
          n204 = case shown="True" w450 {
            frame False {
            }
            frame True {
              n205 = call "Shutdown VI.vi"() -> ()  [unwired: 12 in]
            }
          }
        }
      }
      frame "K2 Failed" {
        (unwired) Cases."Test Failed" ("Enum in")
        n206 = local write "Tab Control"(T10."Page 8" ("Tab Control")) -> ()
        n207 = property on="EXIT Button" class="Bool (strict)"("DisabledEnum"=T5."Enabled" ("Disabled")) -> ()  [unwired: 2 in, 2 out]
        n208 = while {
          stop <- "OK Button 10" stop-if-true
          n209 = local read "EXIT Button"() -> (w455:bool)
          n210 = case shown="True" w455 {
            frame False {
            }
            frame True {
              n211 = call "Shutdown VI.vi"() -> ()  [unwired: 12 in]
            }
          }
        }
      }
      frame "LEDs Failed" {
        n212 = local write "Tab Control"(T1."Page 19" ("Tab Control")) -> ()
        n213 = property on="EXIT Button" class="Bool (strict)"("DisabledEnum"=T5."Enabled" ("Disabled")) -> ()  [unwired: 2 in, 2 out]
        n214 = while {
          stop <- "OK Button 12" stop-if-true
          n215 = local read "EXIT Button"() -> (w458:bool)
          n216 = case shown="True" w458 {
            frame False {
            }
            frame True {
              n217 = call "Shutdown VI.vi"() -> ()  [unwired: 12 in]
            }
          }
        }
      }
    }
  }
